vi "UHR-Fleezers Control (host) - 10.5.vi"() -> ()   [LabVIEW 2010] (continued)
        n1545 = Read from Binary File(5:0.0, 8:w6935, 9:T38."big-endian, network order" ("byte order (0:big-endian, network order)"), 10:-1 ("count (1)"), 11:w6941) -> (0:w6934:errorcluster, 2:w6932:dbl[], 3:w6937:refnum<file>)  [unwired: 2 out]
        n1546 = Array To Cluster(array=w6932) -> (cluster=w6931:T48)
        n1547 = Unbundle(w6931) -> ("[0]"=w6930:dbl, "[1]"=w6929:dbl, "[2]"=w6928:dbl, "[3]"=w6927:dbl, "[4]"=w6926:dbl, "[5]"=w6925:dbl)
        n1548 = Close File(refnum=w6937, error in=w6934) -> (error out=→"Read cal error":errorcluster)  [unwired: 1 out]
        n1549 = Multiply(x=w6925, y=w6922) -> (x*y=w6923:dbl)
        n1550 = local write "T2 kappa_x (pN/nm)"(w6927) -> ()
        n1551 = local write "T1 kappa_x (pN/nm)"(w6928) -> ()
        n1552 = local write "T1 alpha_x (nm/V)"(w6930) -> ()
        n1553 = local write "T2 alpha_x (nm/V)"(w6929) -> ()
        n1554 = Multiply(x=w6926, y=w6922) -> (x*y=w6924:dbl)
        n1555 = local write "T1 offset_x (mV)"(w6924) -> ()
        n1556 = local write "T2 offset_x (mV)"(w6923) -> ()
      }
      event "Abort MCL Scan": Value Change {
        n1557 = event-data() -> ()  [unwired: 7 out]
        n1558 = local write "MCL Scanning"(FALSE ("MCL Scanning")) -> ()
        n1559 = xnode "Read/Write Control"("FPGA VI Reference In"=w6955, "error in"=w6954, "Abort scan (MCL)"="Abort MCL Scan") -> ("error out"=w6953:errorcluster)  [unwired: 1 out]
      }
      event "Update Count (MCL)": Value Change {
        n1560 = event-data() -> ()  [unwired: 7 out]
        n1561 = xnode "Read/Write Control"("FPGA VI Reference In"=w6997, "error in"=w6996, "MCL count"="Update Count (MCL)") -> ("error out"=w6995:errorcluster)  [unwired: 1 out]
      }
      event "Phase adjust (MCL)", "+ phase (MCL)", "- phase (MCL)": Value Change {
        n1562 = event-data() -> ()  [unwired: 7 out]
        n1563 = Negate(x="Phase adjust (MCL)") -> (-x=w7043:i16)
        n1564 = Select(t=w7043, s="- phase (MCL)", f="Phase adjust (MCL)") -> (s? t:f=w7041:i16)
        n1565 = Or(x="- phase (MCL)", y="+ phase (MCL)") -> (x .or. y?=w7036:bool)
        n1566 = xnode "Read/Write Control"("FPGA VI Reference In"=w7045, "error in"=w7044, "Phase count adjustment (MCL)"=w7041) -> ("FPGA VI Reference Out"=w7037:T20, "error out"=w7038:errorcluster)
        n1567 = xnode "Read/Write Control"("FPGA VI Reference In"=w7037, "error in"=w7038, "+ phase (MCL)"=w7036) -> ("error out"=w7035:errorcluster)  [unwired: 1 out]
      }
      event "Abort AOD Scan": Value Change {
        n1568 = event-data() -> ()  [unwired: 7 out]
        n1569 = xnode "Read/Write Control"("FPGA VI Reference In"=w7124, "error in"=w7123, "Abort scan"="Abort AOD Scan") -> ("error out"=w7122:errorcluster)  [unwired: 1 out]
      }
      event "Continuous AOD Scanning": Value Change {
        n1570 = event-data() -> ()  [unwired: 7 out]
        n1571 = xnode "Read/Write Control"("FPGA VI Reference In"=w7166, "error in"=w7165, "Cont. Scan"="Continuous AOD Scanning") -> ("error out"=w7164:errorcluster)  [unwired: 1 out]
      }
      event "Index": Value Change {
        n1572 = event-data() -> ()  [unwired: 7 out]
        n1573 = call "Create new save file.vi"("Insert"="", "Ext"=".dat" ("string"), "Index In"="Index") -> ("Path Out"=→"Save file name":path, "Index Out"=w7205:dbl)
        "Save index" <- w7205
        n1574 = local write "Index"(w7205) -> ()
      }
      event "AO1", "AO2": Value Change {
        w7220 = 10.0 ("y")
        w7219 = 32767.0 ("y")
        n1575 = event-data() -> ()  [unwired: 7 out]
        n1576 = local read "AO2"() -> (w7218:dbl)
        n1577 = local read "AO1"() -> (w7215:dbl)
        n1578 = Multiply(x=w7215, y=w7219) -> (x*y=w7214:dbl)
        n1579 = Multiply(x=w7218, y=w7219) -> (x*y=w7217:dbl)
        n1580 = Divide(x=w7214, y=w7220) -> (x/y=w7213:dbl)
        n1581 = Divide(x=w7217, y=w7220) -> (x/y=w7216:dbl)
        n1582 = To Word Integer(number=w7213) -> (16bit integer=w7221:i16)
        n1583 = To Word Integer(number=w7216) -> (16bit integer=w7222:i16)
        n1584 = xnode "Read/Write Control"("FPGA VI Reference In"=w7212, "error in"=w7211, "AO1"=w7221, "AO2"=w7222) -> ("error out"=w7210:errorcluster)  [unwired: 1 out]
      }
      event "Inject Pump 1": Value Change {
        n1585 = event-data() -> ()  [unwired: 7 out]
        n1586 = disable-structure shown="Disabled" {
          frame Disabled {
            n1587 = local read "Chemyx Syringe Pump Serial Port"() -> (w7280:refnum<visa-resource-name>)
            n1588 = local read "Pump write delay (ms)"() -> (w7281:dbl)
            n1589 = case shown="True" "Inject Pump 1" {
              tunnel: w7281 -> [w7288 w7302]
              tunnel: w7280 -> [w7285 w7301]
              frame False {
                n1590 = flat-sequence {
                  tunnel: w7285 -> [w7289]
                  tunnel: [w7289] -> w7286
                  tunnel: w7288 -> [_]
                  tunnel: [w7292] -> w7287
                  tunnel: w7286 -> [w7292]
                  tunnel: w7287 -> [w7293]
                  tunnel: [w7293] -> w7283
                  tunnel: [w7295] -> w7284
                  tunnel: w7283 -> [w7295]
                  tunnel: w7284 -> [w7297]
                  frame #0 {
                    n1591 = call "Write to pump.vi"("string"="enter pump1", "VISA resource name"=w7289) -> ()  [unwired: 1 out]
                  }
                  frame #1 {
                    n1592 = Wait (ms)(milliseconds to wait="Pump pause delay (ms)") -> ()  [unwired: 1 out]
                  }
                  frame #2 {
                    n1593 = call "Write to pump.vi"("string"="stop", "VISA resource name"=w7293) -> ()  [unwired: 1 out]
                  }
                  frame #3 {
                    n1594 = Wait (ms)(milliseconds to wait=u32 500) -> ()  [unwired: 1 out]
                  }
                  frame #4 {
                    n1595 = call "Write to pump.vi"("string"="stop", "VISA resource name"=w7297) -> ()  [unwired: 1 out]
                  }
                }
              }
              frame True {
                n1596 = flat-sequence {
                  tunnel: w7301 -> [w7311]
                  tunnel: w7302 -> [w7306]
                  tunnel: w7302 -> [w7313]
                  tunnel: w7301 -> [w7314]
                  tunnel: [w7314] -> w7299
                  tunnel: [w7316] -> w7300
                  tunnel: w7299 -> [w7316]
                  tunnel: w7300 -> [w7318]
                  frame #0 {
                    n1597 = local read "All Pump Parameters"() -> (w7305:T6)
                    n1598 = Unbundle By Name(w7305) -> ("Pump 1"=w7312:T49)
                    n1599 = call "Set pump parameters.vi"("Pump write delay (ms)"=w7306, "Volume (uL)"="Ch 2 Inject Volume (uL)", "Rate (uL/h)"="Ch 1 Inject Rate (ul/h)", "Units"=4.0, "Pump #"=1.0, "Pump Parameters In"=w7312, "VISA resource name"=w7311) -> ("Pump Parameters Out"=w7304:T49)  [unwired: 3 in]
                    n1600 = Bundle By Name(cluster=w7305, "Pump 1"=w7304) -> (w7303:T6)
                    n1601 = local write "All Pump Parameters"(w7303) -> ()
                  }
                  frame #1 {
                    n1602 = Wait (ms)(milliseconds to wait=w7313) -> ()  [unwired: 1 out]
                  }
                  frame #2 {
                    n1603 = call "Write to pump.vi"("string"="start", "VISA resource name"=w7314) -> ()  [unwired: 1 out]
                  }
                  frame #3 {
                    n1604 = Wait (ms)(milliseconds to wait=u32 500) -> ()  [unwired: 1 out]
                  }
                  frame #4 {
                    n1605 = call "Write to pump.vi"("string"="start", "VISA resource name"=w7318) -> ()  [unwired: 1 out]
                  }
                }
              }
            }
          }
          frame Enabled {
          }
        }
      }
      event "Inject Pump 3": Value Change {
        n1606 = event-data() -> ()  [unwired: 7 out]
        n1607 = disable-structure shown="Disabled" {
          frame Disabled {
            n1608 = local read "Pump write delay (ms)"() -> (w7321:dbl)
            n1609 = case shown="False" "Inject Pump 3" {
              tunnel: w7321 -> [w7328 w7342]
              tunnel: "Chemyx Syringe Pump Serial Port" -> [w7325 w7341]
              frame False {
                n1610 = flat-sequence {
                  tunnel: w7325 -> [w7329]
                  tunnel: [w7329] -> w7326
                  tunnel: w7328 -> [_]
                  tunnel: [w7332] -> w7327
                  tunnel: w7326 -> [w7332]
                  tunnel: w7327 -> [w7333]
                  tunnel: [w7333] -> w7323
                  tunnel: [w7335] -> w7324
                  tunnel: w7323 -> [w7335]
                  tunnel: w7324 -> [w7337]
                  frame #0 {
                    n1611 = call "Write to pump.vi"("string"="enter pump3", "VISA resource name"=w7329) -> ()  [unwired: 1 out]
                  }
                  frame #1 {
                    n1612 = local read "Pump pause delay (ms)"() -> (w7331:u32)
                    n1613 = Wait (ms)(milliseconds to wait=w7331) -> ()  [unwired: 1 out]
                  }
                  frame #2 {
                    n1614 = call "Write to pump.vi"("string"="stop", "VISA resource name"=w7333) -> ()  [unwired: 1 out]
                  }
                  frame #3 {
                    n1615 = Wait (ms)(milliseconds to wait=u32 0) -> ()  [unwired: 1 out]
                  }
                  frame #4 {
                    n1616 = call "Write to pump.vi"("string"="stop", "VISA resource name"=w7337) -> ()  [unwired: 1 out]
                  }
                }
              }
              frame True {
                n1617 = flat-sequence {
                  tunnel: w7341 -> [w7351]
                  tunnel: w7342 -> [w7346]
                  tunnel: w7342 -> [w7353]
                  tunnel: w7341 -> [w7354]
                  tunnel: [w7354] -> w7339
                  tunnel: [w7357] -> w7340
                  tunnel: w7339 -> [w7357]
                  tunnel: w7340 -> [w7358]
                  frame #0 {
                    n1618 = local read "All Pump Parameters"() -> (w7345:T6)
                    n1619 = Unbundle By Name(w7345) -> ("Pump 3"=w7352:T49)
                    n1620 = call "Set pump parameters.vi"("Pump write delay (ms)"=w7346, "Volume (uL)"="Ch 3 Inject Volume (uL)", "Rate (uL/h)"="Ch 3 Inject Rate (ul/h)", "Units"=4.0, "Pump #"=3.0, "Pump Parameters In"=w7352, "VISA resource name"=w7351) -> ("Pump Parameters Out"=w7344:T49)  [unwired: 3 in]
                    n1621 = Bundle By Name(cluster=w7345, "Pump 3"=w7344) -> (w7343:T6)
                    n1622 = local write "All Pump Parameters"(w7343) -> ()
                  }
                  frame #1 {
                    n1623 = Wait (ms)(milliseconds to wait=w7353) -> ()  [unwired: 1 out]
                  }
                  frame #2 {
                    n1624 = call "Write to pump.vi"("string"="start", "VISA resource name"=w7354) -> ()  [unwired: 1 out]
                  }
                  frame #3 {
                    n1625 = Wait (ms)(milliseconds to wait=u32 500) -> ()  [unwired: 1 out]
                  }
                  frame #4 {
                    n1626 = call "Write to pump.vi"("string"="start", "VISA resource name"=w7358) -> ()  [unwired: 1 out]
                  }
                }
              }
            }
          }
          frame Enabled {
          }
        }
      }
      event "Inject Pump 2": Value Change {
        n1627 = event-data() -> ()  [unwired: 7 out]
        n1628 = disable-structure shown="Disabled" {
          frame Disabled {
            n1629 = local read "Pump write delay (ms)"() -> (w7362:dbl)
            n1630 = flat-sequence {
              tunnel: w7360 -> [w7375]
              tunnel: w7362 -> [w7371]
              tunnel: "Inject Pump 2" -> [_]
              tunnel: w7362 -> [w7377]
              tunnel: w7360 -> [w7378]
              frame #0 {
                n1631 = local read "All Pump Parameters"() -> (w7370:T6)
                n1632 = Multiply(x=60.0, y="Flush Center Ch Rate (ul/m)") -> (x*y=w7367:dbl)
                n1633 = Unbundle By Name(w7370) -> ("Pump 2"=w7376:T49)
                n1634 = call "Set pump parameters.vi"("Pump write delay (ms)"=w7371, "Volume (uL)"="Flush Center Ch Volume (uL)", "Rate (uL/h)"=w7367, "Units"=3.0, "Pump #"=2.0, "Pump Parameters In"=w7376, "VISA resource name"=w7375) -> ("Pump Parameters Out"=w7369:T49)  [unwired: 3 in]
                n1635 = Bundle By Name(cluster=w7370, "Pump 2"=w7369) -> (w7368:T6)
                n1636 = local write "All Pump Parameters"(w7368) -> ()
                n1637 = Add(x="Flush Center Ch Volume (uL)", y="Total Volume\nFlushed (uL)") -> (x+y=w7364:dbl)
                n1638 = local write "Total Volume\nFlushed (uL)"(w7364) -> ()
              }
              frame #1 {
                n1639 = Wait (ms)(milliseconds to wait=w7377) -> ()  [unwired: 1 out]
              }
              frame #2 {
                n1640 = call "Write to pump.vi"("string"="start", "VISA resource name"=w7378) -> ()  [unwired: 1 out]
              }
            }
            n1641 = local read "Chemyx Syringe Pump Serial Port"() -> (w7360:refnum<visa-resource-name>)
          }
          frame Enabled {
          }
        }
      }
      event "Sample Channel Flow": Value Change {
        n1642 = event-data() -> ()  [unwired: 7 out]
        n1643 = Select(t="run" ("string"), s="Sample Channel Flow", f="stop" ("string")) -> (s? t:f=w7380:string)
        n1644 = Concatenate Strings(w7380, "\r") -> (w7384:string)
        n1645 = VISA Write(VISA resource name=w7386, write buffer=w7384) -> ()  [unwired: 1 in, 3 out]
      }
      event "Flip Green Filter": Value Change {
        n1646 = event-data() -> ()  [unwired: 7 out]
        n1647 = Not(x="Flip Green Filter") -> (.not. x?=w7387:bool)
        n1648 = local write "Flip Green Filter"(w7387) -> ()
        n1649 = flat-sequence {
          tunnel: w7395 -> [w7400]
          tunnel: w7394 -> [w7399]
          tunnel: [w7397] -> w7392
          tunnel: [w7396] -> w7391
          tunnel: [w7440] -> w7390
          tunnel: w7392 -> [w7440]
          tunnel: [w7439] -> w7389
          tunnel: w7391 -> [w7439]
          tunnel: w7390 -> [w7444]
          tunnel: w7389 -> [w7443]
          tunnel: [w7442] -> w7393
          frame #0 {
            n1650 = xnode "Read/Write Control"("FPGA VI Reference In"=w7400, "error in"=w7399, "Green Filter Flipper"=TRUE) -> ("FPGA VI Reference Out"=w7397:T20, "error out"=w7396:errorcluster)
          }
          frame #1 {
            n1651 = Wait (ms)(milliseconds to wait=u32 100) -> ()  [unwired: 1 out]
          }
          frame #2 {
            n1652 = xnode "Read/Write Control"("FPGA VI Reference In"=w7444, "error in"=w7443, "Green Filter Flipper"=FALSE) -> ("error out"=w7442:errorcluster)  [unwired: 1 out]
          }
        }
      }
      event "Pump 1 contents", "Pump 3 contents": Value Change {
        n1653 = event-data() -> ()  [unwired: 7 out]
        n1654 = local read "Pump 1 contents"() -> (→"Pump 1 cont disp":string)
        n1655 = local read "Pump 3 contents"() -> (→"Pump 3 cont disp":string)
      }
      event "Reset Trap Pos. FB": Value Change {
        n1656 = event-data() -> ()  [unwired: 7 out]
        n1657 = xnode "Read/Write Control"("FPGA VI Reference In"=w7488, "error in"=w7487, "Trap Pos. FB Reset"="Reset Trap Pos. FB") -> ()  [unwired: 2 out]
      }
      event "Trap Pos. FB ON": Value Change {
        n1658 = event-data() -> ()  [unwired: 7 out]
        n1659 = xnode "Read/Write Control"("FPGA VI Reference In"=w7529, "error in"=w7528, "Force feedback"="Trap Pos. FB ON") -> ()  [unwired: 2 out]
      }
      event "Trap Pos. FB Range", "Trap Pos. FB Gains", "Trap Pos. FB Mult Factor", "Trap Pos. FB Offset Factor", "Trap Pos FB Negate Action", "Trap Pos FB Monitor\nT1 or T2": Value Change {
        n1660 = event-data() -> ()  [unwired: 7 out]
        n1661 = xnode "Read/Write Control"("FPGA VI Reference In"=w7576, "error in"=w7575, "Trap Pos. FB Range"="Trap Pos. FB Range", "Trap Pos. FB Gains"="Trap Pos. FB Gains", "Trap Pos. FB Mult Factor"="Trap Pos. FB Mult Factor", "Trap Pos. FB Offset Factor"="Trap Pos. FB Offset Factor", "Trap Pos FB Negate Action"="Trap Pos FB Negate Action", "Trap Pos FB Monitor T1 or T2"="Trap Pos FB Monitor\nT1 or T2", "AI1 X Scale"="Trap Pos. AI1 X Pre-scale") -> ()  [unwired: 2 out]
      }
      event "Trap Pos FB SP": Value Change {
        n1662 = event-data() -> ()  [unwired: 7 out]
        n1663 = xnode "Read/Write Control"("FPGA VI Reference In"=w7764, "error in"=w7763, "Trap Pos. FB SP"="Trap Pos FB SP") -> ()  [unwired: 2 out]
      }
      event "Set SP to Reading": Value Change {
        n1664 = event-data() -> ()  [unwired: 7 out]
        n1665 = local read "Trap Pos FB Monitor\nT1 or T2"() -> (w7817:bool)
        n1666 = local read "Trap X AI1 (DMA)"() -> (w7820:T14)
        n1667 = local read "Trap X (AI1)"() -> (w7823:T11)
        n1668 = Unbundle By Name(w7823) -> ("Trap 1"=w7822:fxp<+/-,16,1>, "Trap 2"=w7821:fxp<+/-,16,1>)
        n1669 = Unbundle By Name(w7820) -> ("Set 1"=w7819:fxp<+/-,16,1>, "Set 2"=w7818:fxp<+/-,16,1>)
        n1670 = Select(t=w7822, s=w7817, f=w7821) -> (s? t:f=w7816:fxp<+/-,16,1>)
        n1671 = Select(t=w7819, s=w7817, f=w7818) -> (s? t:f=w7815:fxp<+/-,16,1>)
        n1672 = Not(x="Set SP Using...") -> (.not. x?=w7810:bool)
        n1673 = Select(t=w7816, s=w7810, f=w7815) -> (s? t:f=w7811:fxp<+/-,16,1>)
        n1674 = xnode "Read/Write Control"("FPGA VI Reference In"=w7813, "error in"=w7812, "Trap Pos. FB SP"=w7811) -> ()  [unwired: 2 out]
        n1675 = local write "Trap Pos FB SP"(w7811) -> ()
      }
      event "Trap Pos. FB Out Scale 2^n": Value Change {
        n1676 = event-data() -> ()  [unwired: 7 out]
        n1677 = Scale By Power Of 2(n="Trap Pos. FB Out Scale 2^n", x=ext 1.0) -> (x*2^n=w7870:ext)
        n1678 = property on="Trap Pos. FB Mult Factor" class="DigNum (strict)"("Val(Sgnl)"=w7870) -> ()  [unwired: 2 in, 2 out]
      }
      event "Trap Pos FB Int Count": Value Change {
        n1679 = event-data() -> ()  [unwired: 7 out]
        n1680 = xnode "Read/Write Control"("FPGA VI Reference In"=w7875, "error in"=w7874, "Trap Pos FB Int Count"="Trap Pos FB Int Count") -> ()  [unwired: 2 out]
      }
    }
    "error out 2" <- w4364
    n1681 = node-c288() -> ()  [unwired: 2 out]
  }
  n1682 = timed-loop "Run Scripts, including: stage motion" {
    timing: w71 -> [_]
    timing-out: [_] -> w70
    tunnel: w56 -> [w7915]
    tunnel: w57 -> [w7914]
    tunnel: w9 -> [_]
    stop <- w7916 stop-if-true
    n1683 = node-c288() -> ()  [unwired: 1 in, 1 out]
    n1684 = event shown="[10] \"Move to Position 1\", \"Move to Position 2\", \"Move to Position 3\", \"Move to Position 4\", \"Move to Position 5\", \"Lower Ch. Cap.\": Value Change" {
      selector: _ -> [_ _ _ _ _ _ _ _ _ _ _ _ _ _ _ _ _]
      dyn-events: _ -> [_ _ _ _ _ _ _ _ _ _ _ _ _ _ _ _ _]
      timeout: 50 -> [_ _ _ _ _ _ _ _ _ _ _ _ _ _ _ _ _]
      tunnel: ["Set Position" "Move to Position" "Move Cap. 1 (DNA Right)" _ "Move Cap. 2 (ADig Left)" _ "Cal/Data Acq. Spot" "Dump Beads" "Dip for Protein" _ _ "Got ADig bead" "Got DNA bead" "Take Stepping Data" _ "Take Detection Laser\nImage" _] -> _
      tunnel: [_ _ _ _ _ _ _ _ _ _ _ _ _ _ _ _ w8344] -> w7916
      tunnel: w7915 -> [_ _ w7957 _ w8020 _ _ _ _ _ _ _ _ _ _ _ _]
      tunnel: w7914 -> [_ _ w7956 _ w8021 _ _ _ _ _ _ _ _ _ _ _ _]
      event "Set Position", "Set Position 2", "Set Position 3", "Set Position 4", "Set Position 5", "Set Position 1": Value Change {
        n1685 = event-data() -> ()  [unwired: 1 in, 5 out]
        n1686 = Build Array("Set Position 1", "Set Position 2", "Set Position 3", "Set Position 4", "Set Position 5") -> (w7935:bool[])
        n1687 = Boolean Array To Number(Boolean array=w7935) -> (number=w7934:u32)
        n1688 = Logarithm Base 2(1:w7934) -> (0:w7926:dbl)
        n1689 = call "CONEX_FUNCTIONAL_GLOBAL.vi"("Command"=T23."GET POS") -> ("Current Position"=w7919:dbl[])  [unwired: 8 in, 2 out]
        n1690 = Decrement(x="Position") -> (x-1=w7924:dbl)
        n1691 = Greater Or Equal?(x=w7926, y=0.0) -> (x >= y?=w7927:bool)
        n1692 = Select(t=w7926, s=w7927, f=w7924) -> (s? t:f=w7923:dbl)
        n1693 = Increment(x=w7923) -> (x+1=w7922:dbl)
        n1694 = Build Array (concatenate)(w7922, w7919) -> (w7921:dbl[])
        n1695 = Replace Array Subset(array="Saved Stage Positions", new element=w7921, index (row)=w7923) -> (w7936:dbl[][])  [unwired: 1 in]
        n1696 = local write "Saved Stage Positions"(w7936) -> ()
      }
      event "Move to Position": Value Change {
        n1697 = event-data() -> ()  [unwired: 1 in, 5 out]
        n1698 = flat-sequence {
          frame #0 {
            n1699 = local read "Position"() -> (w7951:dbl)
            n1700 = local read "Saved Stage Positions"() -> (w7949:dbl[][])
            n1701 = Decrement(x=w7951) -> (x-1=w7948:dbl)
            n1702 = Array Subset(array=w7949, index (row)=w7948, length (row)=1 ("length"), index (col)=1 ("index"), length (col)=3 ("length")) -> (w7945:dbl[][])
            n1703 = Reshape Array(w7945, 3 ("dimension size")) -> (w7941:dbl[])
            n1704 = local write "Stage Moving"(TRUE ("Stage Moving")) -> ()
            n1705 = call "CONEX_FUNCTIONAL_GLOBAL.vi"("Axis"=enum16{"X", "Y", "Z", "XY", "XZ", "YZ", "XYZ"}."XYZ", "Position"=w7941, "Command"=T23."ABS MOVE") -> ()  [unwired: 6 in, 3 out]
          }
          frame #1 {
            n1706 = call <vilib>:"Beep.vi"() -> ()  [unwired: 3 in, 9 out]
            n1707 = local write "Stage Moving"(FALSE ("Stage Moving")) -> ()
          }
        }
      }
      event "Move Cap. 1 (DNA Right)": Value Change {
        n1708 = event-data() -> ()  [unwired: 1 in, 5 out]
        n1709 = local write "Move Cap. 1 (DNA Right)"(FALSE ("Move Cap. 1 (DNA Right)")) -> ()
        n1710 = flat-sequence {
          tunnel: w7957 -> [w7967]
          tunnel: w7956 -> [w7966]
          tunnel: [w7965] -> w7955
          tunnel: [w7964] -> w7954
          tunnel: ["Cap 1 Samp Flow ON"] -> w7953
          tunnel: w7955 -> [w7987]
          tunnel: w7954 -> [w7986]
          tunnel: w7953 -> [w7985]
          frame #0 {
            n1711 = local read "Saved Stage Positions"() -> (w7974:dbl[][])
            n1712 = Array Subset(array=w7974, index (row)=0 ("index"), length (row)=1 ("length"), index (col)=1 ("index"), length (col)=3 ("length")) -> (w7971:dbl[][])
            n1713 = Reshape Array(w7971, 3 ("dimension size")) -> (w7961:dbl[])
            n1714 = case shown="True" "Cap 1 Samp Flow ON" {
              tunnel: w7966 -> [w7976 w7982]
              tunnel: w7967 -> [w7977 w7981]
              tunnel: [w7977 w7979] -> w7965
              tunnel: [w7976 w7978] -> w7964
              frame False {
              }
              frame True {
                # "run flow"
                n1715 = Concatenate Strings("run" ("string"), "\r") -> (w7983:string)
                n1716 = VISA Write(VISA resource name=w7981, write buffer=w7983, error in (no error)=w7982) -> (VISA resource name out=w7979:refnum<visa-resource-name>, error out=w7978:errorcluster)  [unwired: 1 out]
              }
            }
            n1717 = call "CONEX_FUNCTIONAL_GLOBAL.vi"("Axis"=enum16{"X", "Y", "Z", "XY", "XZ", "YZ", "XYZ"}."XYZ", "Position"=w7961, "Command"=T23."ABS MOVE") -> ()  [unwired: 6 in, 3 out]
            n1718 = local write "Stage Moving"(TRUE ("Stage Moving")) -> ()
          }
          frame #1 {
            n1719 = local write "Stage Moving"(FALSE ("Stage Moving")) -> ()
            n1720 = case shown="True" w7985 {
              tunnel: w7986 -> [w7992 w7998]
              tunnel: w7987 -> [w7993 w7997]
              tunnel: [w7993 w7995] -> _
              tunnel: [w7992 w7994] -> _
              frame False {
              }
              frame True {
                n1721 = Concatenate Strings("stop" ("string"), "\r") -> (w7999:string)
                n1722 = VISA Write(VISA resource name=w7997, write buffer=w7999, error in (no error)=w7998) -> (VISA resource name out=w7995:refnum<visa-resource-name>, error out=w7994:errorcluster)  [unwired: 1 out]
              }
            }
            n1723 = case shown="True" TRUE {
              tunnel: "Cap 1 T ON" -> [w8002 w8003]
              frame False {
                n1724 = property on="Trap 1 (ON/OFF)" class="Bool (strict)"("Val(Sgnl)"=w8002) -> ()  [unwired: 2 in, 2 out]
              }
              frame True {
                n1725 = property on="Trap 2 (ON/OFF)" class="Bool (strict)"("Val(Sgnl)"=w8003) -> ()  [unwired: 2 in, 2 out]
              }
            }
            n1726 = call <vilib>:"Beep.vi"() -> ()  [unwired: 3 in, 9 out]
            n1727 = case shown="True" "Cap 1 Flow ON" {
              frame False {
              }
              frame True {
                n1728 = property on="Inject Pump 1" class="Bool (strict)"("Val(Sgnl)"=TRUE ("Value (Signaling)")) -> ()  [unwired: 2 in, 2 out]
              }
            }
          }
        }
      }
      event Timeout {
        n1729 = event-data() -> ()  [unwired: 1 in, 2 out]
        n1730 = case shown="True" "reset motor comm. link" {
          tunnel: [_ w8010] -> w8004
          frame False {
          }
          frame True {
            n1731 = call "CONEX_FUNCTIONAL_GLOBAL.vi"("Command"=T23."CLOSE") -> ("error out"=w8012:errorcluster)  [unwired: 8 in, 2 out]
            n1732 = flat-sequence {
              tunnel: w8012 -> [w8015]
              tunnel: [w8015] -> w8011
              frame #0 {
                n1733 = Wait (ms)(milliseconds to wait=u32 50) -> ()  [unwired: 1 out]
              }
            }
            n1734 = call "CONEX_FUNCTIONAL_GLOBAL.vi"("error in"=w8011, "Command"=T23."INIT") -> ("error out"=w8010:errorcluster)  [unwired: 7 in, 2 out]
          }
        }
        n1735 = call "CONEX_FUNCTIONAL_GLOBAL.vi"("Axis"=enum16{"X", "Y", "Z", "XY", "XZ", "YZ", "XYZ"}."XYZ", "error in"=w8004, "Command"=T23."GET POS") -> ("Current Position"=w8007:dbl[])  [unwired: 6 in, 2 out]
        n1736 = Array To Cluster(array=w8007) -> (cluster=→"Waveform Chart":T5)
        n1737 = local write "Current Position"(w8007) -> ()
      }
      event "Move Cap. 2 (ADig Left)": Value Change {
        n1738 = event-data() -> ()  [unwired: 1 in, 5 out]
        n1739 = local write "Move Cap. 2 (ADig Left)"(FALSE ("Move Cap. 2 (ADig Left)")) -> ()
        n1740 = flat-sequence {
          tunnel: w8021 -> [w8031]
          tunnel: w8020 -> [w8030]
          tunnel: [w8029] -> w8019
          tunnel: [w8028] -> w8018
          tunnel: ["Cap 2 Samp Flow ON"] -> w8017
          tunnel: w8019 -> [w8051]
          tunnel: w8018 -> [w8050]
          tunnel: w8017 -> [w8049]
          frame #0 {
            n1741 = local read "Saved Stage Positions"() -> (w8038:dbl[][])
            n1742 = case shown="True" "Cap 2 Samp Flow ON" {
              tunnel: w8031 -> [w8040 w8046]
              tunnel: w8030 -> [w8041 w8045]
              tunnel: [w8041 w8043] -> w8029
              tunnel: [w8040 w8042] -> w8028
              frame False {
              }
              frame True {
                # "run flow"
                n1743 = Concatenate Strings("run" ("string"), "\r") -> (w8047:string)
                n1744 = VISA Write(VISA resource name=w8045, write buffer=w8047, error in (no error)=w8046) -> (VISA resource name out=w8043:refnum<visa-resource-name>, error out=w8042:errorcluster)  [unwired: 1 out]
              }
            }
            n1745 = Array Subset(array=w8038, index (row)=1 ("index"), length (row)=1 ("length"), index (col)=1 ("index"), length (col)=3 ("length")) -> (w8035:dbl[][])
            n1746 = Reshape Array(w8035, 3 ("dimension size")) -> (w8025:dbl[])
            n1747 = local write "Stage Moving"(TRUE ("Stage Moving")) -> ()
            n1748 = call "CONEX_FUNCTIONAL_GLOBAL.vi"("Axis"=enum16{"X", "Y", "Z", "XY", "XZ", "YZ", "XYZ"}."XYZ", "Position"=w8025, "Command"=T23."ABS MOVE") -> ()  [unwired: 6 in, 3 out]
          }
          frame #1 {
            n1749 = local write "Stage Moving"(FALSE ("Stage Moving")) -> ()
            n1750 = case shown="True" TRUE {
              tunnel: "Cap 2 T ON" -> [w8062 w8063]
              frame False {
                n1751 = property on="Trap 2 (ON/OFF)" class="Bool (strict)"("Val(Sgnl)"=w8062) -> ()  [unwired: 2 in, 2 out]
              }
              frame True {
                n1752 = property on="Trap 1 (ON/OFF)" class="Bool (strict)"("Val(Sgnl)"=w8063) -> ()  [unwired: 2 in, 2 out]
              }
            }
            n1753 = call <vilib>:"Beep.vi"() -> ()  [unwired: 3 in, 9 out]
            n1754 = case shown="True" w8049 {
              tunnel: w8051 -> [_ w8057]
              tunnel: w8050 -> [_ w8056]
              frame False {
              }
              frame True {
                n1755 = Concatenate Strings("stop" ("string"), "\r") -> (w8059:string)
                n1756 = VISA Write(VISA resource name=w8057, write buffer=w8059, error in (no error)=w8056) -> ()  [unwired: 3 out]
              }
            }
            n1757 = case shown="True" "Cap 2 Flow ON" {
              frame False {
              }
              frame True {
                n1758 = property on="Inject Pump 3" class="Bool (strict)"("Val(Sgnl)"=TRUE ("Value (Signaling)")) -> ()  [unwired: 2 in, 2 out]
              }
            }
          }
        }
      }
      event "+z", "-z": Value Change {
        n1759 = event-data() -> ()  [unwired: 1 in, 5 out]
        n1760 = flat-sequence {
          frame #0 {
            w8065 = 0.0 ("element")
            n1761 = Divide(x="z nudge increment (um)", y=1000.0) -> (x/y=w8078:dbl)
            n1762 = Boolean To (0,1)(Boolean="+z") -> (0, 1=w8071:i16)
            n1763 = Boolean To (0,1)(Boolean="-z") -> (0, 1=w8072:i16)
            n1764 = Multiply(x=w8071, y=w8078) -> (x*y=w8075:dbl)
            n1765 = Multiply(x=w8072, y=w8078) -> (x*y=w8073:dbl)
            n1766 = Negate(x=w8073) -> (-x=w8074:dbl)
            n1767 = Add(x=w8075, y=w8074) -> (x+y=w8066:dbl)
            n1768 = Build Array(w8065, w8065, w8066) -> (w8064:dbl[])
            n1769 = call "CONEX_FUNCTIONAL_GLOBAL.vi"("Axis"=enum16{"X", "Y", "Z", "XY", "XZ", "YZ", "XYZ"}."Z", "Position"=w8064, "Command"=T23."REL MOVE") -> ()  [unwired: 6 in, 3 out]
            n1770 = local write "Stage Moving"(TRUE ("Stage Moving")) -> ()
          }
          frame #1 {
            n1771 = local write "Stage Moving"(FALSE ("Stage Moving")) -> ()
            n1772 = call <vilib>:"Beep.vi"() -> ()  [unwired: 3 in, 9 out]
          }
        }
      }
      event "Cal/Data Acq. Spot": Value Change {
        # "CHANGE FISH FOR TETHER BACK\nTO TRUE VALUE HERE."
        n1773 = event-data() -> ()  [unwired: 1 in, 5 out]
        n1774 = flat-sequence {
          tunnel: ["Cal @ (MHz)"] -> w8081
          tunnel: w8081 -> [w8103]
          tunnel: w8081 -> [w8124]
          frame #0 {
            n1775 = local read "Saved Stage Positions"() -> (w8089:dbl[][])
            n1776 = Array Subset(array=w8089, index (row)=2 ("index"), length (row)=1 ("length"), index (col)=1 ("index"), length (col)=3 ("length")) -> (w8092:dbl[][])
            n1777 = Reshape Array(w8092, 3 ("dimension size")) -> (w8085:dbl[])
            n1778 = local write "Stage Moving"(TRUE ("Stage Moving")) -> ()
            n1779 = call "CONEX_FUNCTIONAL_GLOBAL.vi"("Axis"=enum16{"X", "Y", "Z", "XY", "XZ", "YZ", "XYZ"}."XYZ", "Position"=w8085, "Command"=T23."ABS MOVE") -> ()  [unwired: 6 in, 3 out]
          }
          frame #1 {
            n1780 = property on="Trap Delta (MHz)" class="DigNum (strict)"("Val(Sgnl)"="Cal @ (MHz)") -> ()  [unwired: 2 in, 2 out]
            n1781 = local write "Stage Moving"(FALSE ("Stage Moving")) -> ()
            n1782 = call <vilib>:"Beep.vi"() -> ()  [unwired: 3 in, 9 out]
          }
          frame #2 {
            n1783 = Wait (ms)(milliseconds to wait=u32 100) -> ()  [unwired: 1 out]
          }
          frame #3 {
            n1784 = property on="Save Calibration" class="Bool (strict)"("Val(Sgnl)"=TRUE ("Value (Signaling)")) -> ()  [unwired: 2 in, 2 out]
          }
          frame #4 {
            n1785 = Wait (ms)(milliseconds to wait=u32 4000) -> ()  [unwired: 1 out]
          }
          frame #5 {
            n1786 = while {
              stop <- w8100 stop-if-true
              n1787 = local read "Saving..."() -> (w8101:bool)
              n1788 = Wait (ms)(milliseconds to wait=u32 100) -> ()  [unwired: 1 out]
              n1789 = Not(x=w8101) -> (.not. x?=w8100:bool)
            }
          }
          frame #6 {
            n1790 = case shown="True" "W/ Offset 1" {
              tunnel: w8103 -> [_ w8105]
              frame False {
              }
              frame True {
                n1791 = stacked-sequence {
                  tunnel: w8105 -> [_ _ _ _ _ _ _ w8122]
                  frame #0 {
                    n1792 = property on="Trap Delta (MHz)" class="DigNum (strict)"("Val(Sgnl)"="Offset 1 Start (MHz)") -> ()  [unwired: 2 in, 2 out]
                    n1793 = Replace Array Subset(array=u32[] [0] ("Index Values"), new element="Offset 1 Set", index=0) -> (w8106:u32[])
                    n1794 = property on="Saved AOD Raster Scan Parameter Sets" class="Arr (strict)"("Index Values"=w8106) -> ()  [unwired: 2 in, 2 out]
                  }
                  frame #1 {
                    n1795 = Wait (ms)(milliseconds to wait=u32 200) -> ()  [unwired: 1 out]
                  }
                  frame #2 {
                    n1796 = property on="Load parameters" class="Bool (strict)"("Val(Sgnl)"=TRUE ("Value (Signaling)")) -> ()  [unwired: 2 in, 2 out]
                  }
                  frame #3 {
                    n1797 = Wait (ms)(milliseconds to wait=u32 200) -> ()  [unwired: 1 out]
                  }
                  frame #4 {
                    n1798 = property on="Trap Raster Scan" class="Bool (strict)"("Val(Sgnl)"=TRUE ("Value (Signaling)")) -> ()  [unwired: 2 in, 2 out]
                  }
                  frame #5 {
                    n1799 = Wait (ms)(milliseconds to wait=u32 2000) -> ()  [unwired: 1 out]
                  }
                  frame #6 {
                    n1800 = while {
                      stop <- w8119 stop-if-true
                      n1801 = local read "Raster Scanning..."() -> (w8121:bool)
                      n1802 = local read "Saving..."() -> (w8117:bool)
                      n1803 = Wait (ms)(milliseconds to wait=u32 100) -> ()  [unwired: 1 out]
                      n1804 = Not(x=w8117) -> (.not. x?=w8116:bool)
                      n1805 = Not(x=w8121) -> (.not. x?=w8118:bool)
                      n1806 = And(x=w8118, y=w8116) -> (x .and. y?=w8119:bool)
                    }
                  }
                  frame #7 {
                    n1807 = property on="Trap Delta (MHz)" class="DigNum (strict)"("Val(Sgnl)"=w8122) -> ()  [unwired: 2 in, 2 out]
                  }
                }
              }
            }
          }
          frame #7 {
            n1808 = local read "Save ave N"() -> (w8123:dbl)
            n1809 = case shown="True" "W/ Offset 2" {
              tunnel: w8124 -> [_ w8130]
              tunnel: w8123 -> [_ w8129]
              frame False {
                n1810 = Multiply(x="Cal read wait (s)", y=u32 1000 ("milliseconds to wait")) -> (x*y=w8127:u32)
                n1811 = Wait (ms)(milliseconds to wait=w8127) -> ()  [unwired: 1 out]
              }
              frame True {
                n1812 = stacked-sequence {
                  tunnel: w8130 -> [_ _ _ _ _ _ _ _ _ w8151 _ _]
                  tunnel: w8129 -> [_ _ _ _ _ _ _ _ _ w8149 _ _]
                  frame #0 {
                    n1813 = property on="Save ave N" class="DigNum (strict)"("Val(Sgnl)"=1.0 ("Value (Signaling)")) -> ()  [unwired: 2 in, 2 out]
                  }
                  frame #1 {
                    n1814 = Wait (ms)(milliseconds to wait=u32 500) -> ()  [unwired: 1 out]
                  }
                  frame #2 {
                    n1815 = property on="Trap Delta (MHz)" class="DigNum (strict)"("Val(Sgnl)"="Offset 2 Start (MHz)") -> ()  [unwired: 2 in, 2 out]
                    n1816 = Replace Array Subset(array=u32[] [0] ("Index Values"), new element="Offset 2 Set", index=0) -> (w8135:u32[])
                    n1817 = property on="Saved AOD Raster Scan Parameter Sets" class="Arr (strict)"("Index Values"=w8135) -> ()  [unwired: 2 in, 2 out]
                  }
                  frame #3 {
                    n1818 = Wait (ms)(milliseconds to wait=u32 500) -> ()  [unwired: 1 out]
                  }
                  frame #4 {
                    n1819 = property on="Load parameters" class="Bool (strict)"("Val(Sgnl)"=TRUE ("Value (Signaling)")) -> ()  [unwired: 2 in, 2 out]
                  }
                  frame #5 {
                    n1820 = Wait (ms)(milliseconds to wait=u32 500) -> ()  [unwired: 1 out]
                  }
                  frame #6 {
                    n1821 = property on="Trap Raster Scan" class="Bool (strict)"("Val(Sgnl)"=TRUE ("Value (Signaling)")) -> ()  [unwired: 2 in, 2 out]
                  }
                  frame #7 {
                    n1822 = Wait (ms)(milliseconds to wait=u32 2000) -> ()  [unwired: 1 out]
                  }
                  frame #8 {
                    n1823 = while {
                      stop <- w8144 stop-if-true
                      n1824 = local read "Raster Scanning..."() -> (w8147:bool)
                      n1825 = local read "Saving..."() -> (w8145:bool)
                      n1826 = Wait (ms)(milliseconds to wait=u32 100) -> ()  [unwired: 1 out]
                      n1827 = Not(x=w8145) -> (.not. x?=w8143:bool)
                      n1828 = Not(x=w8147) -> (.not. x?=w8146:bool)
                      n1829 = And(x=w8146, y=w8143) -> (x .and. y?=w8144:bool)
                    }
                  }
                  frame #9 {
                    n1830 = property on="Trap Delta (MHz)" class="DigNum (strict)"("Val(Sgnl)"=w8151) -> ()  [unwired: 2 in, 2 out]
                    n1831 = property on="Saved AOD Raster Scan Parameter Sets" class="Arr (strict)"("Index Values"=u32[] [0]) -> ()  [unwired: 2 in, 2 out]
                    n1832 = property on="Save ave N" class="DigNum (strict)"("Val(Sgnl)"=w8149) -> ()  [unwired: 2 in, 2 out]
                  }
                  frame #10 {
                    n1833 = Wait (ms)(milliseconds to wait=u32 500) -> ()  [unwired: 1 out]
                  }
                  frame #11 {
                    n1834 = property on="Load parameters" class="Bool (strict)"("Val(Sgnl)"=TRUE ("Value (Signaling)")) -> ()  [unwired: 2 in, 2 out]
                  }
                }
              }
            }
          }
          frame #8 {
            n1835 = property on="Read Cal" class="Bool (strict)"("Val(Sgnl)"=TRUE ("Value (Signaling)")) -> ()  [unwired: 2 in, 2 out]
          }
          frame #9 {
            n1836 = Wait (ms)(milliseconds to wait=u32 500) -> ()  [unwired: 1 out]
          }
          frame #10 {
            n1837 = property on="Fish for Tether" class="Bool (strict)"("Val(Sgnl)"=FALSE ("Value (Signaling)")) -> ()  [unwired: 2 in, 2 out]
          }
        }
        n1838 = local write "Cal/Data Acq. Spot"(FALSE ("Cal/Data Acq. Spot")) -> ()
      }
      event "Dump Beads": Value Change {
        # "SCRIPT TO REMOVE BOTH BEADS FROM THE TRAPS. TURNS ON LIGHT WHICH INDICATES THAT STAGE IS MOVING. THEN STOPS SAVING DATA. \nSETS Sample Channel Flow TO TRUE. STOPS INTERLACING GREEN FLUORESCENCE. TURNS OFF Tether INDICATOR BECAUSE WE ARE THROWING IT\nAWAY. SHUTS OFF TRAP POSITION FEEDBACK."
        n1839 = event-data() -> ()  [unwired: 1 in, 5 out]
        n1840 = flat-sequence {
          frame #0 {
            w8158 = FALSE ("Fl. Triggered...")
            w8159 = TRUE ("Stage Moving")
            n1841 = local read "Saving..."() -> (w8160:bool)
            n1842 = local write "Fl. Triggered..."(w8158) -> ()
            n1843 = local write "Stage Moving"(w8159) -> ()
            n1844 = local write "Tether"(w8158) -> ()
            n1845 = property on="Green Laser ON/Interlacing" class="Bool (strict)"("Val(Sgnl)"=w8158) -> ()  [unwired: 2 in, 2 out]
            n1846 = property on="Trap Pos. FB ON" class="Bool (strict)"("Val(Sgnl)"=w8158) -> ()  [unwired: 2 in, 2 out]
            n1847 = property on="Sample Channel Flow" class="Bool (strict)"("Val(Sgnl)"=w8159) -> ()  [unwired: 2 in, 2 out]
            n1848 = local write "Stop Saving"(w8160) -> ()
          }
          frame #1 {
            # "MOVES TO THE DUMP BEADS POSITION"
            n1849 = local read "Saved Stage Positions"() -> (w8164:dbl[][])
            n1850 = Array Subset(array=w8164, index (row)=3 ("index"), length (row)=1 ("length"), index (col)=1 ("index"), length (col)=3 ("length")) -> (w8167:dbl[][])
            n1851 = Reshape Array(w8167, 3 ("dimension size")) -> (w8162:dbl[])
            n1852 = call "CONEX_FUNCTIONAL_GLOBAL.vi"("Axis"=enum16{"X", "Y", "Z", "XY", "XZ", "YZ", "XYZ"}."XYZ", "Position"=w8162, "Command"=T23."ABS MOVE") -> ()  [unwired: 6 in, 3 out]
          }
          frame #2 {
            w8171 = FALSE ("Value (Signaling)")
            # "TURNS TRAPS OFF SO THAT\nBEADS REMAIN AT DUMP \nBEADS POSITION"
            n1853 = property on="Trap 1 (ON/OFF)" class="Bool (strict)"("Val(Sgnl)"=w8171) -> ()  [unwired: 2 in, 2 out]
            n1854 = property on="Trap 2 (ON/OFF)" class="Bool (strict)"("Val(Sgnl)"=w8171) -> ()  [unwired: 2 in, 2 out]
            n1855 = call <vilib>:"Beep.vi"() -> ()  [unwired: 3 in, 9 out]
          }
          frame #3 {
            # "MOVES STAGE BACK TO THE\nANTIDIG CAPILARY BY CALLING\nTHE Move Cap. 2 SCRIPT"
            n1856 = property on="Move Cap. 2 (ADig Left)" class="Bool (strict)"("Val(Sgnl)"=TRUE ("Value (Signaling)")) -> ()  [unwired: 2 in, 2 out]
          }
        }
      }
      event "Dip for Protein": Value Change {
        n1857 = event-data() -> ()  [unwired: 1 in, 5 out]
        n1858 = flat-sequence {
          frame #0 {
            n1859 = case shown="True" "Move Trap Before?" {
              frame False {
              }
              frame True {
                n1860 = property on="Trap Delta (MHz)" class="DigNum (strict)"("Val(Sgnl)"="Dip Trap Delta 1 (MHz)") -> ()  [unwired: 2 in, 2 out]
              }
            }
          }
          frame #1 {
            n1861 = local read "Saved Stage Positions"() -> (w8179:dbl[][])
            n1862 = Array Subset(array=w8179, index (row)=4 ("index"), length (row)=1 ("length"), index (col)=1 ("index"), length (col)=3 ("length")) -> (w8182:dbl[][])
            n1863 = Reshape Array(w8182, 3 ("dimension size")) -> (w8177:dbl[])
            n1864 = call "CONEX_FUNCTIONAL_GLOBAL.vi"("Axis"=enum16{"X", "Y", "Z", "XY", "XZ", "YZ", "XYZ"}."XYZ", "Position"=w8177, "Command"=T23."ABS MOVE") -> ()  [unwired: 6 in, 3 out]
          }
          frame #2 {
            n1865 = Multiply(x="Duration (s)", y=1000.0) -> (x*y=w8186:dbl)
            n1866 = Wait (ms)(milliseconds to wait=w8186) -> ()  [unwired: 1 out]
          }
          frame #3 {
            n1867 = local read "Saved Stage Positions"() -> (w8192:dbl[][])
            n1868 = Array Subset(array=w8192, index (row)=2 ("index"), length (row)=1 ("length"), index (col)=1 ("index"), length (col)=3 ("length")) -> (w8195:dbl[][])
            n1869 = Reshape Array(w8195, 3 ("dimension size")) -> (w8190:dbl[])
            n1870 = call "CONEX_FUNCTIONAL_GLOBAL.vi"("Axis"=enum16{"X", "Y", "Z", "XY", "XZ", "YZ", "XYZ"}."XYZ", "Position"=w8190, "Command"=T23."ABS MOVE") -> ()  [unwired: 6 in, 3 out]
          }
          frame #4 {
            n1871 = case shown="True" "Move Trap After?" {
              frame False {
              }
              frame True {
                n1872 = property on="Trap Delta (MHz)" class="DigNum (strict)"("Val(Sgnl)"="Dip Trap Delta 2 (MHz)") -> ()  [unwired: 2 in, 2 out]
              }
            }
          }
          frame #5 {
            n1873 = case shown="True" "Green ON After?" {
              frame False {
              }
              frame True {
                n1874 = property on="Green Laser ON/Interlacing" class="Bool (strict)"("Val(Sgnl)"=TRUE ("Value (Signaling)")) -> ()  [unwired: 2 in, 2 out]
              }
            }
          }
          frame #6 {
            n1875 = Wait (ms)(milliseconds to wait=u32 500) -> ()  [unwired: 1 out]
          }
          frame #7 {
            n1876 = case shown="True" "Save Data After?" {
              frame False {
              }
              frame True {
                n1877 = property on="Start Saving" class="Bool (strict)"("Val(Sgnl)"=TRUE ("Value (Signaling)")) -> ()  [unwired: 2 in, 2 out]
              }
            }
          }
        }
      }
      event "Profile": Value Change {
        n1878 = event-data() -> ()  [unwired: 1 in, 5 out]
        n1879 = flat-sequence {
          tunnel: [w8208] -> w8207
          tunnel: w8207 -> [w8212]
          tunnel: [w8211] -> w8206
          tunnel: w8206 -> [w8218]
          frame #0 {
            w8209 = 0.0 ("element")
            n1880 = Build Array(w8209, "Y change (mm)", w8209) -> (w8208:dbl[])
          }
          frame #1 {
            # "move to new position and start saving"
            n1881 = local write "Stage Moving"(TRUE ("Stage Moving")) -> ()
            n1882 = local write "Start Saving"(TRUE ("Start Saving")) -> ()
            n1883 = call "CONEX_FUNCTIONAL_GLOBAL.vi"("Axis"=enum16{"X", "Y", "Z", "XY", "XZ", "YZ", "XYZ"}."Y", "Position"=w8212, "Command"=T23."REL MOVE") -> ()  [unwired: 6 in, 3 out]
            n1884 = Negate(x=w8212) -> (-x=w8211:dbl[])
          }
          frame #2 {
            # "go back to start"
            n1885 = call "CONEX_FUNCTIONAL_GLOBAL.vi"("Axis"=enum16{"X", "Y", "Z", "XY", "XZ", "YZ", "XYZ"}."Y", "Position"=w8218, "Command"=T23."REL MOVE") -> ()  [unwired: 6 in, 3 out]
          }
          frame #3 {
            # "stop saving"
            n1886 = local write "Stop Saving"(TRUE ("Stop Saving")) -> ()
            n1887 = local write "Stage Moving"(FALSE ("Stage Moving")) -> ()
          }
        }
      }
      event "Move to Position 1", "Move to Position 2", "Move to Position 3", "Move to Position 4", "Move to Position 5", "Lower Ch. Cap.": Value Change {
        n1888 = event-data() -> ()  [unwired: 1 in, 5 out]
        n1889 = Or(x="Move to Position 5", y="Lower Ch. Cap.") -> (x .or. y?=w8223:bool)
        n1890 = Build Array("Move to Position 1", "Move to Position 2", "Move to Position 3", "Move to Position 4", w8223) -> (w8226:bool[])
        n1891 = Boolean Array To Number(Boolean array=w8226) -> (number=w8225:u32)
        n1892 = Logarithm Base 2(1:w8225) -> (0:w8224:dbl)
        n1893 = flat-sequence {
          tunnel: w8224 -> [w8236]
          frame #0 {
            n1894 = local read "Saved Stage Positions"() -> (w8241:dbl[][])
            n1895 = Array Subset(array=w8241, index (row)=w8236, length (row)=1 ("length"), index (col)=1 ("index"), length (col)=3 ("length")) -> (w8238:dbl[][])
            n1896 = Reshape Array(w8238, 3 ("dimension size")) -> (w8233:dbl[])
            n1897 = local write "Stage Moving"(TRUE ("Stage Moving")) -> ()
            n1898 = call "CONEX_FUNCTIONAL_GLOBAL.vi"("Axis"=enum16{"X", "Y", "Z", "XY", "XZ", "YZ", "XYZ"}."XYZ", "Position"=w8233, "Command"=T23."ABS MOVE") -> ()  [unwired: 6 in, 3 out]
          }
          frame #1 {
            n1899 = local write "Stage Moving"(FALSE ("Stage Moving")) -> ()
            n1900 = call <vilib>:"Beep.vi"() -> ()  [unwired: 3 in, 9 out]
          }
        }
      }
      event "Got ADig bead": Value Change {
        n1901 = event-data() -> ()  [unwired: 1 in, 5 out]
        n1902 = property on="Move Cap. 1 (DNA Right)" class="Bool (strict)"("Val(Sgnl)"=TRUE ("Value (Signaling)")) -> ()  [unwired: 2 in, 2 out]
        n1903 = property on="Inject Pump 3" class="Bool (strict)"("Val(Sgnl)"=FALSE ("Value (Signaling)")) -> ()  [unwired: 2 in, 2 out]
      }
      event "Got DNA bead": Value Change {
        n1904 = event-data() -> ()  [unwired: 1 in, 5 out]
        n1905 = property on="Cal/Data Acq. Spot" class="Bool (strict)"("Val(Sgnl)"=TRUE ("Value (Signaling)")) -> ()  [unwired: 2 in, 2 out]
        n1906 = property on="Inject Pump 1" class="Bool (strict)"("Val(Sgnl)"=FALSE ("Value (Signaling)")) -> ()  [unwired: 2 in, 2 out]
      }
      event "Take Stepping Data": Value Change {
        n1907 = event-data() -> ()  [unwired: 1 in, 5 out]
        n1908 = local read "Save ave N"() -> (w8258:dbl)
        n1909 = flat-sequence {
          tunnel: w8258 -> [w8260]
          tunnel: [w8260] -> w8253
          tunnel: [w8262] -> w8254
          tunnel: w8253 -> [w8262]
          tunnel: [w8264] -> w8255
          tunnel: w8254 -> [w8264]
          tunnel: [w8267] -> w8256
          tunnel: w8255 -> [w8267]
          tunnel: [w8269] -> w8257
          tunnel: w8256 -> [w8269]
          tunnel: [w8271] -> w8251
          tunnel: w8257 -> [w8271]
          tunnel: w8251 -> [w8274]
          tunnel: [w8274] -> w8250
          tunnel: w8250 -> [w8275]
          tunnel: [w8275] -> w8252
          tunnel: w8252 -> [w8281]
          frame #0 {
            n1910 = property on="Save ave N" class="DigNum (strict)"("Val(Sgnl)"="Save ave factor") -> ()  [unwired: 2 in, 2 out]
          }
          frame #1 {
            n1911 = Wait (ms)(milliseconds to wait=u32 100) -> ()  [unwired: 1 out]
          }
          frame #2 {
            n1912 = local read "Offset 2 Start (MHz)"() -> (w8266:dbl)
            n1913 = property on="Saved AOD Raster Scan Parameter Sets" class="Arr (strict)"("Index Values"=u32[] [2]) -> ()  [unwired: 2 in, 2 out]
            n1914 = property on="Trap Delta (MHz)" class="DigNum (strict)"("Val(Sgnl)"=w8266) -> ()  [unwired: 2 in, 2 out]
          }
          frame #3 {
            n1915 = property on="Load parameters" class="Bool (strict)"("Val(Sgnl)"=TRUE ("Value (Signaling)")) -> ()  [unwired: 2 in, 2 out]
          }
          frame #4 {
            n1916 = Wait (ms)(milliseconds to wait=u32 100) -> ()  [unwired: 1 out]
          }
          frame #5 {
            n1917 = property on="Trap Raster Scan" class="Bool (strict)"("Val(Sgnl)"=TRUE ("Value (Signaling)")) -> ()  [unwired: 2 in, 2 out]
          }
          frame #6 {
            n1918 = Wait (ms)(milliseconds to wait=u32 1000) -> ()  [unwired: 1 out]
          }
          frame #7 {
            n1919 = while {
              stop <- w8278 stop-if-true
              n1920 = local read "Raster Scanning..."() -> (w8280:bool)
              n1921 = local read "Saving..."() -> (w8279:bool)
              n1922 = Not(x=w8279) -> (.not. x?=w8276:bool)
              n1923 = Not(x=w8280) -> (.not. x?=w8277:bool)
              n1924 = And(x=w8277, y=w8276) -> (x .and. y?=w8278:bool)
            }
          }
          frame #8 {
            n1925 = property on="Save ave N" class="DigNum (strict)"("Val(Sgnl)"=w8281) -> ()  [unwired: 2 in, 2 out]
          }
        }
      }
      event "Step Size (nm)": Value Change {
        n1926 = event-data() -> ()  [unwired: 1 in, 5 out]
        n1927 = flat-sequence {
          frame #0 {
            n1928 = property on="Saved AOD Raster Scan Parameter Sets" class="Arr (strict)"("Index Values"=u32[] [1]) -> ()  [unwired: 2 in, 2 out]
          }
          frame #1 {
            n1929 = Multiply(x="N Steps", y="Step Size (nm)") -> (x*y=w8283:dbl)
            n1930 = property on="Scan Speed AOD (nm/s) 2" class="DigNum (strict)"("Value"="Step Size (nm)") -> ()  [unwired: 2 in, 2 out]
            n1931 = property on="Step Size AOD (nm) 2" class="DigNum (strict)"("Value"="Step Size (nm)") -> ()  [unwired: 2 in, 2 out]
            n1932 = property on="Scan Range AOD (nm) 2" class="DigNum (strict)"("Value"=w8283) -> ()  [unwired: 2 in, 2 out]
          }
        }
      }
      event "Take Detection Laser\nImage": Value Change {
        n1933 = event-data() -> ()  [unwired: 1 in, 5 out]
        n1934 = flat-sequence {
          tunnel: [w8311] -> w8301
          tunnel: [w8310] -> w8294
          tunnel: [w8309] -> w8286
          tunnel: [w8314] -> w8302
          tunnel: w8301 -> [w8314]
          tunnel: [w8313] -> w8295
          tunnel: w8294 -> [w8313]
          tunnel: [w8312] -> w8287
          tunnel: w8286 -> [w8312]
          tunnel: [w8318] -> w8303
          tunnel: w8302 -> [w8318]
          tunnel: [w8317] -> w8296
          tunnel: w8295 -> [w8317]
          tunnel: [w8316] -> w8288
          tunnel: w8287 -> [w8316]
          tunnel: [w8324] -> w8304
          tunnel: w8303 -> [w8324]
          tunnel: [w8323] -> w8297
          tunnel: w8296 -> [w8323]
          tunnel: [w8322] -> w8289
          tunnel: w8288 -> [w8322]
          tunnel: [w8328] -> w8305
          tunnel: w8304 -> [w8328]
          tunnel: [w8327] -> w8298
          tunnel: w8297 -> [w8327]
          tunnel: [w8326] -> w8290
          tunnel: w8289 -> [w8326]
          tunnel: [w8332] -> w8306
          tunnel: w8305 -> [w8332]
          tunnel: [w8331] -> w8299
          tunnel: w8298 -> [w8331]
          tunnel: [w8330] -> w8291
          tunnel: w8290 -> [w8330]
          tunnel: [w8336] -> w8307
          tunnel: w8306 -> [w8336]
          tunnel: [w8335] -> w8300
          tunnel: w8299 -> [w8335]
          tunnel: [w8334] -> w8292
          tunnel: w8291 -> [w8334]
          tunnel: w8307 -> [w8342]
          tunnel: w8300 -> [w8341]
          tunnel: [w8339] -> w8293
          tunnel: w8292 -> [w8339]
          tunnel: w8293 -> [w8343]
          frame #0 {
            n1935 = local read "Green Laser ON/Interlacing"() -> (w8311:bool)
            n1936 = local read "Green laser mode"() -> (w8310:enum32{"Laser ON", "Laser OFF", "Interlace"})
            n1937 = local read "Green FB On/Off"() -> (w8309:bool)
          }
          frame #1 {
            n1938 = property on="Green FB On/Off" class="Bool (strict)"("Val(Sgnl)"=FALSE ("Value (Signaling)")) -> ()  [unwired: 2 in, 2 out]
          }
          frame #2 {
            n1939 = property on="Green Laser ON/Interlacing" class="Bool (strict)"("Val(Sgnl)"=TRUE ("Value (Signaling)")) -> ()  [unwired: 2 in, 2 out]
            n1940 = property on="Flip Green Filter" class="Bool (strict)"("Val(Sgnl)"=TRUE ("Value (Signaling)")) -> ()  [unwired: 2 in, 2 out]